vi "Transpose intensity graph.vi"() -> ()   [LabVIEW 2016]
panel:
  out "Derivative of Data 2":dbl[][](graph)
  in  "Derivative of Data":dbl[][](graph)=array1215x321[390015 elements]
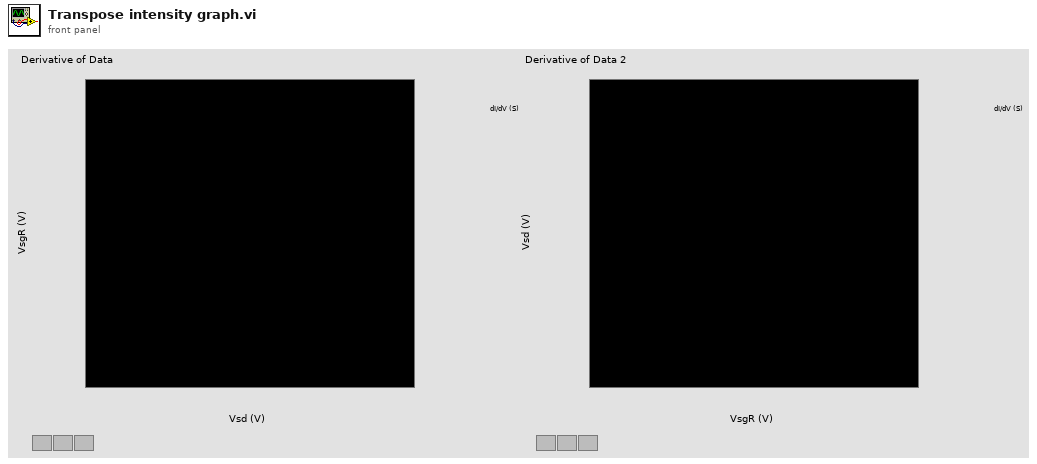
[diagram p1: front panel]
types:
  T1 = typedef "LVOffsetAndMultiplierTypeDef.ctl" = cluster{"Offset":dbl, "Multiplier":dbl}
  T2 = typedef "LVRangeTypeDef.ctl" = cluster{"Minimum":dbl, "Maximum":dbl, "Increment":dbl, "Minor Increment":dbl, "Start":dbl}
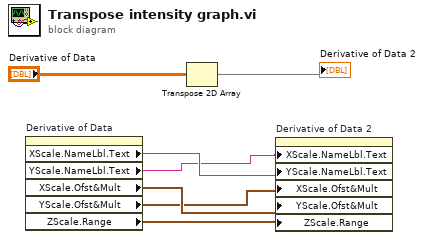
[diagram p0: block diagram]
diagram:
  n1 = property on="Derivative of Data" class="IntGraph (strict)"() -> ("XScale.NameLbl.Text"=w5:string, "YScale.NameLbl.Text"=w4:string, "XScale.Ofst&Mult"=w3:T1, "YScale.Ofst&Mult"=w2:T1, "ZScale.Range"=w1:T2)  [unwired: 2 in, 2 out]
  n2 = Transpose 2D Array(2D array="Derivative of Data") -> (transposed array=→"Derivative of Data 2":dbl[][])
  n3 = property on="Derivative of Data 2" class="IntGraph (strict)"("XScale.NameLbl.Text"=w4, "YScale.NameLbl.Text"=w5, "XScale.Ofst&Mult"=w2, "YScale.Ofst&Mult"=w3, "ZScale.Range"=w1) -> ()  [unwired: 2 in, 2 out]
